vi "HFRR ADV v042.vi"() -> ()   [LabVIEW 2025] (continued)
                  }
                  frame True {
                    n297 = Not(x=w407) -> (.not. x?=w406:bool)
                    n298 = call "ELAPSED TIMER VI - abort test.vi"("TARGET"=60.0, "RESET"=w406, "PAUSE"=FALSE) -> ("ELAPSED INDICATION"=w404:bool)  [unwired: 6 in, 2 out]
                    n299 = case shown="True" w404 {
                      frame False {
                      }
                      frame True {
                        n300 = stacked-sequence {
                          frame #0 {
                            w409 = FALSE
                            n301 = local write "RUN"(w409) -> ()
                            n302 = local write "Auto Start Test"(w409) -> ()
                          }
                          frame #1 {
                            n303 = One Button Dialog(message="Test stopped due to a communication error. Reconnect the C1 and C2 cables.") -> ()  [unwired: 1 in, 1 out]
                          }
                        }
                      }
                    }
                  }
                }
              }
            }
          }
          frame Enabled {
          }
        }
        n304 = Get Date/Time In Seconds() -> (seconds since 1Jan1904=w390:timestamp)
        n305 = Format Into String(format string="%<%I:%M:%S:%p %d:%B:%Y>T", w390) -> (resulting string=→"Time Stamp":string)  [unwired: 2 in, 1 out]
        n306 = local read "Service Password enable"() -> (w382:bool)
        n307 = local read "FILE"() -> (w387:string)
        n308 = call <vilib>:"Trim Whitespace.vi"("string"=w387) -> ("trimmed string"=w386:string)  [unwired: 1 in]
        n309 = String Length(string=w386) -> (length=w385:i32)
        n310 = Greater?(x=w385, y=1) -> (0:w383:bool)
        n311 = case shown="False" w383 {
          tunnel: w382 -> [w411 _]
          frame False {
            n312 = case shown="False" w411 {
              frame True {
                w412 = "Test Start In Service Mode" ("Tip Strip")
                w413 = T19."Enabled" ("Disabled")
                n313 = property on="Auto Start Test" class="Bool (strict)"("DisabledEnum"=w413, "TipStrip"=w412) -> ()  [unwired: 2 in, 2 out]
                n314 = property on="RUN" class="Bool (strict)"("DisabledEnum"=w413, "TipStrip"=w412) -> ()  [unwired: 2 in, 2 out]
              }
              frame False {
                w414 = "Enter File Name to Start Test" ("Tip Strip")
                w415 = T19."Disabled and Grayed Out" ("Disabled")
                n315 = property on="Auto Start Test" class="Bool (strict)"("DisabledEnum"=w415, "TipStrip"=w414) -> ()  [unwired: 2 in, 2 out]
                n316 = property on="RUN" class="Bool (strict)"("DisabledEnum"=w415, "TipStrip"=w414) -> ()  [unwired: 2 in, 2 out]
              }
            }
          }
          frame True {
            w416 = "" ("Tip Strip")
            w417 = T19."Enabled" ("Disabled")
            n317 = property on="Auto Start Test" class="Bool (strict)"("DisabledEnum"=w417, "TipStrip"=w416) -> ()  [unwired: 2 in, 2 out]
            n318 = property on="RUN" class="Bool (strict)"("DisabledEnum"=w417, "TipStrip"=w416) -> ()  [unwired: 2 in, 2 out]
          }
        }
      }
      event "RUN": Value Change {
        n319 = event-data() -> ()  [unwired: 1 in, 6 out]
        n320 = local read "RUN"() -> (w419:bool)
        n321 = case shown="False" w419 {
          frame False {
            n322 = flat-sequence {
              frame #0 {
                n323 = local write "START TEMP"(FALSE ("START TEMP")) -> ()
              }
              frame #1 {
                n324 = Wait (ms)(milliseconds to wait=u32 1500) -> ()  [unwired: 1 out]
              }
              frame #2 {
                n325 = local write "Humidity 2"(TRUE ("Humidity")) -> ()
              }
              frame #3 {
                n326 = local write "Due Write"("VC;0") -> ()
              }
              frame #4 {
                n327 = Wait (ms)(milliseconds to wait=u32 1500) -> ()  [unwired: 1 out]
              }
              frame #5 {
                w429 = T19."Enabled" ("Disabled")
                (unwired) T25."Imaging" ("Main Dashboard Buttons")
                (unwired) T21."Adv Scar" ("Main Tab")
                w431 = "" ("FILE")
                n328 = local write "measured_stroke"(0.0 ("measured_stroke")) -> ()
                n329 = local write "Due Write"("VC;0") -> ()
                n330 = local write "FILE"(w431) -> ()
                n331 = local write "Batch Ref Num :"(w431) -> ()
                n332 = local write "Fuel Discription :"(w431) -> ()
                n333 = local write "Main Tab"(T2."Adv Scar" ("Main Tab")) -> ()
                n334 = local write "Remarks :"(w431) -> ()
                n335 = local write "Main Dashboard Buttons"(T1."Imaging" ("Main Dashboard Buttons")) -> ()
                n336 = local write "TEST FILE NAM,E SAVED"(FALSE ("TEST FILE NAM,E SAVED")) -> ()
                n337 = property on="Stroke ( mm )" class="WFChart (strict)"("History Data"=cluster{"y":dbl, dbl, "y":dbl}[] []) -> ()  [unwired: 2 in, 2 out]
                n338 = property on="Auto Start Test" class="Bool (strict)"("Visible"=TRUE) -> ()  [unwired: 2 in, 2 out]
                n339 = property on="FRICVALZ 2" class="Bool (strict)"("DisabledEnum"=w429) -> ()  [unwired: 2 in, 2 out]
                n340 = property on="FRICVALZ 4" class="Bool (strict)"("DisabledEnum"=w429) -> ()  [unwired: 2 in, 2 out]
                n341 = property on="FRICVALZ 3" class="Bool (strict)"("DisabledEnum"=w429) -> ()  [unwired: 2 in, 2 out]
              }
            }
          }
          frame True {
            n342 = stacked-sequence {
              frame #0 {
                n343 = local write "Due Write"("DAC;200") -> ()
              }
              frame #1 {
                n344 = Wait (ms)(milliseconds to wait=u32 1500) -> ()  [unwired: 1 out]
              }
              frame #2 {
                n345 = local write "Due Write"("DAC;200") -> ()
              }
              frame #3 {
                n346 = Wait (ms)(milliseconds to wait=u32 1500) -> ()  [unwired: 1 out]
              }
              frame #4 {
                n347 = local write "Due Write"("VC;1") -> ()
              }
              frame #5 {
                n348 = Wait (ms)(milliseconds to wait=u32 2000) -> ()  [unwired: 1 out]
              }
              frame #6 {
                n349 = local write "Due Write"("VC;1") -> ()
              }
              frame #7 {
                n350 = Wait (ms)(milliseconds to wait=u32 2000) -> ()  [unwired: 1 out]
              }
              frame #8 {
                w443 = T19."Disabled" ("Disabled")
                n351 = property on="Auto Start Test" class="Bool (strict)"("Visible"=FALSE) -> ()  [unwired: 2 in, 2 out]
                n352 = local write "START TEMP"(TRUE ("START TEMP")) -> ()
                n353 = property on="FRICVALZ 2" class="Bool (strict)"("DisabledEnum"=w443) -> ()  [unwired: 2 in, 2 out]
                n354 = property on="FRICVALZ 4" class="Bool (strict)"("DisabledEnum"=w443) -> ()  [unwired: 2 in, 2 out]
                n355 = property on="FRICVALZ 3" class="Bool (strict)"("DisabledEnum"=w443) -> ()  [unwired: 2 in, 2 out]
              }
            }
          }
        }
      }
      event "run test Calibration": Value Change {
        n356 = event-data() -> ()  [unwired: 1 in, 6 out]
        n357 = local read "run test Calibration"() -> (w445:bool)
        n358 = case shown="True" w445 {
          frame False {
            n359 = flat-sequence {
              frame #0 {
                n360 = local write "START TEMP"(FALSE ("START TEMP")) -> ()
              }
              frame #1 {
                n361 = Wait (ms)(milliseconds to wait=u32 1500) -> ()  [unwired: 1 out]
              }
              frame #2 {
              }
              frame #3 {
                n362 = local write "Due Write"("VC;0") -> ()
              }
              frame #4 {
                n363 = Wait (ms)(milliseconds to wait=u32 1500) -> ()  [unwired: 1 out]
              }
              frame #5 {
                n364 = local write "Due Write"("VC;0") -> ()
                n365 = local write "Friction Force Calibration Result Tab"(enum32{"Calibration Results", "Page 2"}."Calibration Results" ("Friction Force Calibration Result Tab")) -> ()
                n366 = property on="Friction Force Calibration Result Tab" class="TabCtl (strict)"("Visible"=TRUE) -> ()  [unwired: 2 in, 2 out]
              }
            }
          }
          frame True {
            n367 = flat-sequence {
              frame #0 {
                n368 = local write "Due Write"("VC;1") -> ()
              }
              frame #1 {
                n369 = Wait (ms)(milliseconds to wait=u32 2000) -> ()  [unwired: 1 out]
              }
              frame #2 {
                n370 = local write "Due Write"("VC;1") -> ()
              }
              frame #3 {
                n371 = Wait (ms)(milliseconds to wait=u32 2000) -> ()  [unwired: 1 out]
              }
              frame #4 {
                n372 = local write "START TEMP"(TRUE ("START TEMP")) -> ()
                n373 = local write "Friction Force Calibration Result Tab"(enum32{"Calibration Results", "Page 2"}."Calibration Results" ("Friction Force Calibration Result Tab")) -> ()
                n374 = property on="Friction Force Calibration Result Tab" class="TabCtl (strict)"("Visible"=TRUE) -> ()  [unwired: 2 in, 2 out]
              }
            }
          }
        }
      }
      event "Auto": Value Change {
        n375 = event-data() -> ()  [unwired: 1 in, 6 out]
        n376 = stacked-sequence {
          frame #0 {
            n377 = local write "FILE"("") -> ()
          }
          frame #1 {
            n378 = Get Date/Time In Seconds() -> (seconds since 1Jan1904=w465:timestamp)
            n379 = Format Into String(format string="%<%I_%M_%S_%p_%d_%B_%Y>T", w465) -> (resulting string=w464:string)  [unwired: 2 in, 1 out]
            n380 = local write "FILE"(w464) -> ()
          }
        }
        n381 = local read "Auto"() -> (w462:bool)
        n382 = Not(x=w462) -> (.not. x?=w461:bool)
        n383 = local write "Auto"(w461) -> ()
      }
      event "Auto Start Temp": Value Change {
        n384 = event-data() -> ()  [unwired: 1 in, 6 out]
        n385 = local read "Auto Start Test"() -> (w468:bool)
        n386 = case shown="False" w468 {
          frame False {
            n387 = stacked-sequence {
              frame #0 {
                n388 = local write "START TEMP"(FALSE ("START TEMP")) -> ()
              }
              frame #1 {
                n389 = Wait (ms)(milliseconds to wait=u32 2000) -> ()  [unwired: 1 out]
              }
              frame #2 {
                n390 = local write "Due Write"("VC;0") -> ()
              }
              frame #3 {
                n391 = Wait (ms)(milliseconds to wait=u32 2000) -> ()  [unwired: 1 out]
              }
              frame #4 {
                w479 = T19."Enabled" ("Disabled")
                (unwired) T25."Imaging" ("Main Dashboard Buttons")
                w480 = "" ("FILE")
                n392 = local write "Main Tab"(T2."Adv Scar" ("Main Tab")) -> ()
                n393 = local write "measured_stroke"(0.0 ("measured_stroke")) -> ()
                n394 = local write "Main Dashboard Buttons"(T1."Imaging" ("Main Dashboard Buttons")) -> ()
                n395 = property on="RUN" class="Bool (strict)"("Visible"=TRUE) -> ()  [unwired: 2 in, 2 out]
                n396 = local write "Due Write"("VC;0") -> ()
                n397 = local write "Humidity 2"(TRUE ("Humidity")) -> ()
                n398 = local write "TEST FILE NAM,E SAVED"(FALSE ("TEST FILE NAM,E SAVED")) -> ()
                n399 = local write "Fuel Discription :"(w480) -> ()
                n400 = local write "Batch Ref Num :"(w480) -> ()
                n401 = local write "Remarks :"(w480) -> ()
                n402 = local write "FILE"(w480) -> ()
                n403 = property on="FRICVALZ 2" class="Bool (strict)"("DisabledEnum"=w479) -> ()  [unwired: 2 in, 2 out]
                n404 = property on="FRICVALZ 4" class="Bool (strict)"("DisabledEnum"=w479) -> ()  [unwired: 2 in, 2 out]
                n405 = property on="FRICVALZ 3" class="Bool (strict)"("DisabledEnum"=w479) -> ()  [unwired: 2 in, 2 out]
              }
            }
          }
          frame True {
            n406 = stacked-sequence {
              frame #0 {
                n407 = local write "Due Write"("DAC;200") -> ()
              }
              frame #1 {
                n408 = Wait (ms)(milliseconds to wait=u32 1500) -> ()  [unwired: 1 out]
              }
              frame #2 {
                n409 = local write "Due Write"("DAC;200") -> ()
              }
              frame #3 {
                n410 = Wait (ms)(milliseconds to wait=u32 1000) -> ()  [unwired: 1 out]
              }
              frame #4 {
                n411 = local write "Due Write"("VC;1") -> ()
              }
              frame #5 {
                n412 = Wait (ms)(milliseconds to wait=u32 2000) -> ()  [unwired: 1 out]
              }
              frame #6 {
                n413 = local write "Due Write"("VC;1") -> ()
              }
              frame #7 {
                n414 = Wait (ms)(milliseconds to wait=u32 2000) -> ()  [unwired: 1 out]
              }
              frame #8 {
                w491 = T19."Disabled" ("Disabled")
                n415 = property on="RUN" class="Bool (strict)"("Visible"=FALSE) -> ()  [unwired: 2 in, 2 out]
                n416 = property on="FRICVALZ 2" class="Bool (strict)"("DisabledEnum"=w491) -> ()  [unwired: 2 in, 2 out]
                n417 = property on="FRICVALZ 4" class="Bool (strict)"("DisabledEnum"=w491) -> ()  [unwired: 2 in, 2 out]
                n418 = property on="FRICVALZ 3" class="Bool (strict)"("DisabledEnum"=w491) -> ()  [unwired: 2 in, 2 out]
                "START TEMP" <- TRUE
              }
            }
          }
        }
      }
      event "FILE", "USERNAME", "USER ID": Mouse Enter {
        n419 = event-data() -> ()  [unwired: 1 in, 4 out]
        n420 = dll-call lib="kernel32.dll" fn="Wow64DisableWow64FsRedirection"("OldValue"=0) -> (error out=w498:errorcluster, "OldValue"=w496:i32)  [unwired: 4 in, 1 out]
        n421 = call <vilib>:"System Exec.vi"("run minimized? (F)"=TRUE, "error in (no error)"=w498, "command line"="C:\\Program Files\\Common Files\\Microsoft Shared\\Ink\\TabTip.exe") -> ("error out"=w497:errorcluster)  [unwired: 5 in, 3 out]
        n422 = dll-call lib="kernel32.dll" fn="Wow64EnableWow64FsRedirection"(error in=w497, "OldValue"=w496) -> ()  [unwired: 4 in, 2 out]
      }
      event "EDIT": Value Change {
        n423 = event-data() -> ()  [unwired: 1 in, 6 out]
        n424 = local read "EDIT"() -> (w499:bool)
        n425 = case shown="False" w499 {
          frame False {
            n426 = control-ref of="This VI"() -> (w516:refnum<vi>)
            n427 = property class="VI"(reference=w516) -> (reference out=w507:refnum<vi>, error out=w511:errorcluster, "Panel"=w515:refnum<vi>)  [unwired: 1 in]
            n428 = property class="Pnl"(reference=w515, error in=w511) -> (reference out=w509:refnum<vi>, error out=w512:errorcluster, "Panes[]"=w514:refnum<vi>[])
            n429 = for {
              tunnel: w514 -> [w522] mode=indexing
              tunnel: T24."Always Off" ("Horizontal Scrollbar Visibility") -> [w521]
              tunnel: w512 -> [w518]
              tunnel: [w517] -> w510
              n430 = property class="Pane"(reference=w522, error in=w518, "HorizScrollbarVisibility"=w521) -> (reference out=w519:refnum<vi>, error out=w520:errorcluster)
              n431 = Close Reference(reference=w519, error in (no error)=w520) -> (error out=w517:errorcluster)
            }
            n432 = Close Reference(reference=w509, error in (no error)=w510) -> (error out=w508:errorcluster)
            n433 = Close Reference(reference=w507, error in (no error)=w508) -> (error out=w502:errorcluster)
            "error out 7" <- w502
            n434 = call <vilib>:"Clear Errors.vi"("error in (no error)"=w502) -> ("error out"=w501:errorcluster)  [unwired: 5 in, 1 out]
            n435 = local write "Service Password enable"(FALSE ("Service Password enable")) -> ()
            n436 = call <userlib>:"Fit VI window to Largest Dec.vi"("error in (no error)"=w501, "border spacing (2 px)"=1) -> ("error out"=w506:errorcluster, "dup VI Ref"=w504:refnum<vi>)  [unwired: 4 in]
            n437 = invoke on="Invoke Node" class="VI" method="FP.Run-Time Position.Maximized"(reference=w504, error in=w506) -> (error out=w505:errorcluster)  [unwired: 2 in, 3 out]
            n438 = call <vilib>:"Clear Errors.vi"("error in (no error)"=w505) -> ()  [unwired: 5 in, 2 out]
          }
          frame True {
          }
        }
      }
      event "Heater Button": Value Change {
        n439 = event-data() -> ()  [unwired: 1 in, 6 out]
        n440 = local read "Heater Button"() -> (w523:bool)
        n441 = case shown="True" w523 {
          frame True {
            n442 = stacked-sequence {
              frame #0 {
                n443 = Wait (ms)(milliseconds to wait=u32 1500) -> ()  [unwired: 1 out]
              }
              frame #1 {
                n444 = local read "Set Temp"() -> (w525:dbl)
                n445 = Number To Fractional String(number=w525, precision (6)=i16 2) -> (F-format string=w528:string)  [unwired: 2 in]
                n446 = Concatenate Strings("ST;" ("Command"), w528) -> (w527:string)
                n447 = local write "Due Write"(w527) -> ()
              }
              frame #2 {
                n448 = Wait (ms)(milliseconds to wait=u32 1500) -> ()  [unwired: 1 out]
              }
              frame #3 {
                n449 = local write "Due Write"("HE;1" ("Command")) -> ()
              }
              frame #4 {
                n450 = Wait (ms)(milliseconds to wait=u32 1500) -> ()  [unwired: 1 out]
              }
              frame #5 {
                n451 = stacked-sequence {
                  frame #0 {
                    n452 = Wait (ms)(milliseconds to wait=u32 1500) -> ()  [unwired: 1 out]
                  }
                  frame #1 {
                    n453 = local read "Set Temp"() -> (w534:dbl)
                    n454 = Number To Fractional String(number=w534, precision (6)=i16 2) -> (F-format string=w537:string)  [unwired: 2 in]
                    n455 = Concatenate Strings("ST;" ("Command"), w537) -> (w536:string)
                    n456 = local write "Due Write"(w536) -> ()
                  }
                  frame #2 {
                    n457 = Wait (ms)(milliseconds to wait=u32 1500) -> ()  [unwired: 1 out]
                  }
                  frame #3 {
                    n458 = local write "Due Write"("HE;1" ("Command")) -> ()
                  }
                  frame #4 {
                    n459 = Wait (ms)(milliseconds to wait=u32 1500) -> ()  [unwired: 1 out]
                  }
                }
              }
            }
          }
          frame False {
            n460 = stacked-sequence {
              frame #0 {
                n461 = Wait (ms)(milliseconds to wait=u32 1500) -> ()  [unwired: 1 out]
              }
              frame #1 {
                n462 = Concatenate Strings("ST;" ("Command"), "0" ("string")) -> (w544:string)
                n463 = local write "Due Write"(w544) -> ()
              }
              frame #2 {
                n464 = Wait (ms)(milliseconds to wait=u32 1500) -> ()  [unwired: 1 out]
              }
              frame #3 {
                n465 = local write "Due Write"("HE;0" ("Command")) -> ()
              }
              frame #4 {
                n466 = Wait (ms)(milliseconds to wait=u32 1500) -> ()  [unwired: 1 out]
              }
            }
          }
        }
      }
      event "Headen Service Button": Value Change {
        n467 = event-data() -> ()  [unwired: 1 in, 6 out]
        n468 = local read "Headen Service Button"() -> (w549:bool)
        n469 = case shown="True" w549 {
          frame False {
            n470 = property on="Password 3" class="Clust (strict)"("Visible"=FALSE) -> ()  [unwired: 2 in, 2 out]
            n471 = property on="Service Password Log" class="Str"("Visible"=FALSE) -> ()  [unwired: 2 in, 2 out]
          }
          frame True {
            n472 = property on="Password 3" class="Clust (strict)"("Visible"=TRUE) -> ()  [unwired: 2 in, 2 out]
            n473 = property on="Service Password Log" class="Str"("Visible"=TRUE) -> ()  [unwired: 2 in, 2 out]
          }
        }
      }
      event "Password 3.Service Password": Value Change {
        n474 = event-data() -> ()  [unwired: 1 in, 6 out]
        n475 = Unbundle By Name("Password 3") -> ("Service Password"=w556:string)
        n476 = call <vilib>:"Trim Whitespace.vi"("string"=w556) -> ("trimmed string"=w554:string)  [unwired: 1 in]
        n477 = Equal?(x=w554, y="Service@123") -> (x = y?=w555:bool)
        n478 = case shown="False" w555 {
          selector: w555 -> [w559 w561]
          frame False {
            n479 = local write "Service Password enable"(w559) -> ()
            n480 = property on="Service Password Log" class="Str"("Visible"=TRUE) -> ()  [unwired: 2 in, 2 out]
          }
          frame True {
            n481 = property on="Service Password Log" class="Str"("Visible"=FALSE) -> ()  [unwired: 2 in, 2 out]
            "Service Password enable" <- w561
          }
        }
      }
      event "Sign In": Value Change {
        w563 = FALSE ("Visible")
        n482 = event-data() -> ()  [unwired: 1 in, 6 out]
        n483 = property on="About" class="Clust (strict)"("Visible"=w563) -> ()  [unwired: 2 in, 2 out]
        n484 = property on="Password 3" class="Clust (strict)"("Visible"=w563) -> ()  [unwired: 2 in, 2 out]
        n485 = property on="Service Password Log" class="Str"("Visible"=FALSE) -> ()  [unwired: 2 in, 2 out]
      }
      event "Info": Value Change {
        n486 = event-data() -> ()  [unwired: 1 in, 6 out]
        n487 = local read "Info"() -> (w565:bool)
        n488 = case shown="False" w565 {
          frame False {
            n489 = property on="About" class="Clust (strict)"("Visible"=FALSE) -> ()  [unwired: 2 in, 2 out]
          }
          frame True {
            n490 = property on="About" class="Clust (strict)"("Visible"=TRUE) -> ()  [unwired: 2 in, 2 out]
          }
        }
      }
      event "Calibration": Value Change {
        n491 = event-data() -> ()  [unwired: 1 in, 6 out]
        n492 = local read "Calibration"() -> (w569:bool)
        n493 = case shown="False" w569 {
          frame False {
            n494 = property on="Calibration 2" class="TabCtl (strict)"("Visible"=FALSE) -> ()  [unwired: 2 in, 2 out]
            n495 = local write "Cal Password"("" ("Cal Password")) -> ()
          }
          frame True {
            n496 = property on="Calibration 2" class="TabCtl (strict)"("Visible"=TRUE) -> ()  [unwired: 2 in, 2 out]
            n497 = local write "Cal Password"("" ("Cal Password")) -> ()
          }
        }
        n498 = property on="Wrong Password" class="Str"("Visible"=FALSE) -> ()  [unwired: 2 in, 2 out]
      }
      event "Cal Password": Value Change {
        n499 = event-data() -> ()  [unwired: 1 in, 6 out]
        n500 = local read "Cal Password"() -> (w577:string)
        n501 = call <vilib>:"Trim Whitespace.vi"("string"=w577) -> ("trimmed string"=w576:string)  [unwired: 1 in]
        n502 = Equal?(x=w576, y="Cal@321") -> (x = y?=w574:bool)
        n503 = case shown="True" w574 {
          frame False {
            n504 = property on="Wrong Password" class="Str"("Visible"=TRUE) -> ()  [unwired: 2 in, 2 out]
          }
          frame True {
            n505 = property on="Wrong Password" class="Str"("Visible"=FALSE) -> ()  [unwired: 2 in, 2 out]
            n506 = local write "Main Tab"(T2."About" ("Main Tab")) -> ()
            n507 = local write "Cal Password"("" ("Cal Password")) -> ()
            n508 = local write "Main Dashboard Buttons"(T1."About" ("Main Dashboard Buttons")) -> ()
            n509 = property on="Calibration 2" class="TabCtl (strict)"("Visible"=FALSE) -> ()  [unwired: 2 in, 2 out]
            n510 = local write "Calibration"(FALSE ("Calibration")) -> ()
          }
        }
      }
      event "Calibration Selection": Value Change {
        n511 = event-data() -> ()  [unwired: 1 in, 6 out]
        n512 = local read "Calibration Selection"() -> (w586:T8)
        n513 = case shown="\"Stroke Calibration\"" w586 {
          tunnel: [T7."Stroke" ("Main Calibration Tab") T7."Friction" ("Main Calibration Tab") T7."Main" ("Main Calibration Tab") T7."Temperature" ("Main Calibration Tab")] -> w585
          frame "Stroke Calibration" {
          }
          frame "Friction Force Calibration" {
          }
          frame Default {
          }
          frame "Temperature Calibration" {
          }
        }
        n514 = local write "Main Calibration Tab"(w585) -> ()
      }
      event "Back Stroke": Value Change {
        n515 = event-data() -> ()  [unwired: 1 in, 6 out]
        n516 = local write "Main Stroke Tab"(T9."Step 1" ("Main Stroke Tab")) -> ()
        n517 = local write "Main Calibration Tab"(T7."Main" ("Main Calibration Tab")) -> ()
        n518 = local write "Back Stroke"(FALSE ("Back Stroke")) -> ()
        n519 = local write "Calibration Selection"(T8."Default" ("Calibration Selection")) -> ()
      }
      event "Step 2 Back": Value Change {
        n520 = event-data() -> ()  [unwired: 1 in, 6 out]
        n521 = local write "Main Stroke Tab"(T9."Step 1" ("Main Stroke Tab")) -> ()
        n522 = local write "Step 2 Back"(FALSE ("Back Stroke")) -> ()
        n523 = local write "Calibration Selection"(T8."Default" ("Calibration Selection")) -> ()
      }
      event "Step 3 Back": Value Change {
        n524 = event-data() -> ()  [unwired: 1 in, 6 out]
        n525 = local write "Main Stroke Tab"(T9."Step 2" ("Main Stroke Tab")) -> ()
        n526 = local write "Step 3 Back"(FALSE ("Back Stroke")) -> ()
        n527 = local write "Calibration Selection"(T8."Default" ("Calibration Selection")) -> ()
      }
      event "Step 4 Back": Value Change {
        n528 = event-data() -> ()  [unwired: 1 in, 6 out]
        n529 = local write "Main Stroke Tab"(T9."Step 3" ("Main Stroke Tab")) -> ()
        n530 = local write "Step 4 Back"(FALSE ("Back Stroke")) -> ()
        n531 = local write "Calibration Selection"(T8."Default" ("Calibration Selection")) -> ()
      }
      event "Step 5 Back": Value Change {
        n532 = event-data() -> ()  [unwired: 1 in, 6 out]
        n533 = local write "Main Stroke Tab"(T9."Step 4" ("Main Stroke Tab")) -> ()
        n534 = local write "Step 5 Back"(FALSE ("Back Stroke")) -> ()
        n535 = local write "Calibration Selection"(T8."Default" ("Calibration Selection")) -> ()
      }
      event "Step 6 Back": Value Change {
        n536 = event-data() -> ()  [unwired: 1 in, 6 out]
        n537 = local write "Main Stroke Tab"(T9."Step 5" ("Main Stroke Tab")) -> ()
        n538 = local write "Step 6 Back"(FALSE ("Back Stroke")) -> ()
        n539 = local write "Calibration Selection"(T8."Default" ("Calibration Selection")) -> ()
      }
      event "Back Stroke step 7": Value Change {
        n540 = event-data() -> ()  [unwired: 1 in, 6 out]
        n541 = local write "Main Stroke Tab"(T9."Step 5" ("Main Stroke Tab")) -> ()
        n542 = local write "Back Stroke step 7"(FALSE ("Back Stroke")) -> ()
        n543 = local write "Calibration Selection"(T8."Default" ("Calibration Selection")) -> ()
      }
      event "Back Stroke step 8": Value Change {
        n544 = event-data() -> ()  [unwired: 1 in, 6 out]
        n545 = local write "Main Stroke Tab"(T9."Step 7" ("Main Stroke Tab")) -> ()
        n546 = local write "Back Stroke step 8"(FALSE ("Back Stroke")) -> ()
        n547 = local write "Calibration Selection"(T8."Default" ("Calibration Selection")) -> ()
      }
      event "Back Stroke 8": Value Change {
        n548 = event-data() -> ()  [unwired: 1 in, 6 out]
        n549 = local write "MOVE CARRIAGE TO"(1.0 ("MOVE CARRIAGE TO")) -> ()
        n550 = local write "Main Stroke Tab"(T9."Step 1" ("Main Stroke Tab")) -> ()
        n551 = local write "Calibration Selection"(T8."Default" ("Calibration Selection")) -> ()
        n552 = local write "Back Stroke 8"(FALSE ("Back Stroke 8")) -> ()
      }
      event "Continue Stroke": Value Change {
        n553 = event-data() -> ()  [unwired: 1 in, 6 out]
        n554 = local write "Main Stroke Tab"(T9."Step 2" ("Main Stroke Tab")) -> ()
        n555 = local write "Continue Stroke"(FALSE ("Continue Stroke")) -> ()
      }
      event "Continue Stroke step 2": Value Change {
        n556 = event-data() -> ()  [unwired: 1 in, 6 out]
        n557 = local write "Main Stroke Tab"(T9."Step 3" ("Main Stroke Tab")) -> ()
        n558 = local write "Continue Stroke step 2"(FALSE ("Continue Stroke")) -> ()
      }
      event "Continue Stroke step 3": Value Change {
        n559 = event-data() -> ()  [unwired: 1 in, 6 out]
        n560 = local write "Main Stroke Tab"(T9."Step 4" ("Main Stroke Tab")) -> ()
        n561 = local write "Continue Stroke step 3"(FALSE ("Continue Stroke")) -> ()
      }
      event "Continue Stroke step 4": Value Change {
        n562 = event-data() -> ()  [unwired: 1 in, 6 out]
        n563 = local write "Main Stroke Tab"(T9."Step 5" ("Main Stroke Tab")) -> ()
        n564 = local write "Continue Stroke step 4"(FALSE ("Continue Stroke")) -> ()
      }
      event "Continue Stroke step 5": Value Change {
        n565 = event-data() -> ()  [unwired: 1 in, 6 out]
        n566 = local write "Main Stroke Tab"(T9."Step 7" ("Main Stroke Tab")) -> ()
        n567 = local write "Continue Stroke step 5"(FALSE ("Continue Stroke")) -> ()
      }
      event "Continue Stroke step 6": Value Change {
        n568 = event-data() -> ()  [unwired: 1 in, 6 out]
        n569 = local write "Main Stroke Tab"(T9."Step 7" ("Main Stroke Tab")) -> ()
        n570 = local write "Continue Stroke step 6"(FALSE ("Continue Stroke")) -> ()
      }
      event "Continue Stroke step 7": Value Change {
        w634 = FALSE ("0.2mm")
        n571 = event-data() -> ()  [unwired: 1 in, 6 out]
        n572 = local write "0.4 mm"(w634) -> ()
        n573 = local write "0.6 mm"(w634) -> ()
        n574 = local write "1.0 mm"(w634) -> ()
        n575 = local write "1.2 mm"(w634) -> ()
        n576 = local write "0.2 2"(w634) -> ()
        n577 = local write "0.4 2"(w634) -> ()
        n578 = local write "0.6 2"(w634) -> ()
        n579 = local write "0.8 2"(w634) -> ()
        n580 = local write "1.0 2"(w634) -> ()
        n581 = local write "1.2"(w634) -> ()
        n582 = local write "0.2mm"(w634) -> ()
        n583 = local write "0.8mm"(w634) -> ()
        n584 = local write "Main Stroke Tab"(T9."Step 8" ("Main Stroke Tab")) -> ()
        n585 = local write "Continue Stroke step 7"(FALSE ("Continue Stroke")) -> ()
        n586 = local write "Stroke Test Complete"(T10."Test Progress" ("Stroke Test Complete")) -> ()
        "Position Measurment Temp" <- 4.0 ("Position Measurment Temp")
        "Calibration Tare" <- TRUE ("Calibration Tare")
        "MOVE CARRIAGE TO" <- 1.0 ("MOVE CARRIAGE TO")
      }
      event "Continue Stroke step 8": Value Change {
        n587 = event-data() -> ()  [unwired: 1 in, 6 out]
        n588 = local read "LVDT STROKE  Calibration"() -> (w639:dbl)
        n589 = local read "Position Measurment Temp"() -> (w640:dbl)
        n590 = case shown="7" w640 {
          selector: w640 -> [w645 w650 w655 w660 _ w668 w671 w672]
          tunnel: w639 -> [w641 w646 w651 w656 w662 w665 _ _]
          frame 0, Default {
            w643 = TRUE ("0.2mm")
            n591 = Increment(x=w645) -> (x+1=w644:i32)
            n592 = local write "Position Measurment Temp"(w644) -> ()
            n593 = local write "0.2mm"(w643) -> ()
            n594 = local write "0.2 2"(w643) -> ()
            n595 = local write "MOVE CARRIAGE TO"(1.0 ("MOVE CARRIAGE TO")) -> ()
            "Calibration 0.2" <- w641
          }
          frame 1 {
            w648 = TRUE ("0.4 mm")
            n596 = Increment(x=w650) -> (x+1=w649:i32)
            n597 = local write "Calibration 0.4"(w646) -> ()
            n598 = local write "Position Measurment Temp"(w649) -> ()
            n599 = local write "0.4 mm"(w648) -> ()
            n600 = local write "MOVE CARRIAGE TO"(0.6 ("MOVE CARRIAGE TO")) -> ()
            n601 = local write "0.4 2"(w648) -> ()
          }
          frame 2 {
            w653 = TRUE ("0.6 mm")
            n602 = Increment(x=w655) -> (x+1=w654:i32)
            n603 = local write "Calibration 0.6"(w651) -> ()
            n604 = local write "Position Measurment Temp"(w654) -> ()
            n605 = local write "0.6 2"(w653) -> ()
            n606 = local write "0.6 mm"(w653) -> ()
            n607 = local write "MOVE CARRIAGE TO"(0.8 ("MOVE CARRIAGE TO")) -> ()
          }
          frame 3 {
            w657 = TRUE ("0.6 mm")
            n608 = Increment(x=w660) -> (x+1=w659:i32)
            n609 = local write "Position Measurment Temp"(w659) -> ()
            n610 = local write "MOVE CARRIAGE TO"(1.0 ("MOVE CARRIAGE TO")) -> ()
            n611 = local write "0.8mm"(w657) -> ()
            n612 = local write "0.8 2"(w657) -> ()
            "Calibration 0.8" <- w656
          }
          frame 4 {
            w663 = TRUE ("0.6 mm")
            n613 = local write "Position Measurment Temp"(6.0 ("Position Measurment Temp")) -> ()
            n614 = local write "MOVE CARRIAGE TO"(1.0 ("MOVE CARRIAGE TO")) -> ()
            n615 = local write "1.0 mm"(w663) -> ()
            n616 = local write "1.0 2"(w663) -> ()
            "Calibration 1.0" <- w662
          }
          frame 5 {
            w666 = TRUE ("0.6 mm")
            n617 = Increment(x=w668) -> (x+1=w667:i32)
            n618 = local write "Position Measurment Temp"(w667) -> ()
            n619 = local write "1.2 mm"(w666) -> ()
            n620 = local write "1.2"(w666) -> ()
            "Calibration 1.2" <- w665
          }
          frame 6 {
            n621 = Increment(x=w671) -> (x+1=w670:i32)
            n622 = local write "Position Measurment Temp"(w670) -> ()
            n623 = local write "Stroke Test Complete"(T10."Stroke Points Completed" ("Stroke Test Complete")) -> ()
          }
          frame 7 {
            n624 = stacked-sequence {
              tunnel: w672 -> [w673 _ _]
              frame #0 {
                n625 = Increment(x=w673) -> (x+1=w674:i32)
                n626 = local write "Main Stroke Tab"(T9."Step 9" ("Main Stroke Tab")) -> ()
                n627 = local write "Position Measurment Temp"(w674) -> ()
                n628 = Insert Into Array(array=dbl[] [], new element #1=0.2 ("new element/subarray"), new element #2=0.4 ("new element/subarray"), new element #3=0.6 ("new element/subarray"), new element #4=0.8 ("new element/subarray"), new element #5=1.0 ("new element/subarray"), new element #6=1.2 ("new element/subarray")) -> (→"1D stroke":dbl[])  [unwired: 1 in]
                n629 = local read "Calibration 0.2"() -> (w681:dbl)
                n630 = local read "Calibration 0.4"() -> (w680:dbl)
                n631 = local read "Calibration 0.6"() -> (w679:dbl)
                n632 = local read "Calibration 0.8"() -> (w678:dbl)
                n633 = local read "Calibration 1.0"() -> (w677:dbl)
                n634 = local read "Calibration 1.2"() -> (w676:dbl)
                n635 = Insert Into Array(array=dbl[] [], new element #1=w681, new element #2=w680, new element #3=w679, new element #4=w678, new element #5=w677, new element #6=w676) -> (→"Calibrated Voltage Value":dbl[])  [unwired: 1 in]
              }
              frame #1 {
                n636 = local read "calibration values"() -> (w704:dbl[])
                n637 = local read "Calibrated Voltage Value"() -> (w706:dbl[])
                n638 = Index Array(array=w704, index #1=1 ("index"), index #2=3 ("index"), index #3=5 ("index"), index #4=7 ("index"), index #5=9 ("index"), index #6=11 ("index")) -> (element #1=w697:dbl, element #2=w696:dbl, element #3=w695:dbl, element #4=w694:dbl, element #5=w693:dbl, element #6=w692:dbl)
                n639 = local read "1D stroke"() -> (w707:dbl[])
                n640 = for {
                  tunnel: [w716] -> w705 mode=indexing
                  tunnel: w707 -> [w715] mode=indexing
                  tunnel: w706 -> [w714] mode=indexing
                  tunnel: w697 -> [w713]
                  tunnel: w696 -> [w712]
                  tunnel: w695 -> [w711]
                  tunnel: w694 -> [w710]
                  tunnel: w693 -> [w709]
                  tunnel: w692 -> [w708]
                  n641 = formula code="if (stroke == 0.2)\n{\n    if ((voltage >= REF_02 - 0.2) && (voltage <= REF_02 + 0.2))\n        status = 1;\n    else\n        status = 0;\n}\nelse if (stroke == 0.4)\n{\n    if ((voltage >= REF_04 - 0.2) && (voltage <= REF_04 + 0.2))\n        status = 1;\n    else\n        status = 0;\n}\nelse if (stroke == 0.6)\n{\n    if ((voltage >= REF_06 - 0.2) && (voltage <= REF_06 + 0.2))\n        status = 1;\n    else\n        status = 0;\n}\nelse if (stroke == 0.8)\n{\n    if ((voltage >= REF_08 - 0.2) && (voltage <= REF_08 + 0.2))\n        status = 1;\n    else\n        status = 0;\n}\nelse if (stroke == 1.0)\n{\n    if ((voltage >= REF_10 - 0.4) && (voltage <= REF_10 + 0.4))\n        status = 1;\n    else\n        status = 0;\n}\nelse if (stroke == 1.2)\n{\n    if ((voltage >= REF_12 - 0.2) && (voltage <= REF_12 + 0.2))\n        status = 1;\n    else\n        status = 0;\n}\nelse\n{\n    status = 0;\n}"("stroke"=w715, "voltage"=w714, "REF_02"=w713, "REF_04"=w712, "REF_06"=w711, "REF_08"=w710, "REF_10"=w709, "REF_12"=w708) -> ("status"=w716:dbl)
                }
                "Status" <- w705
              }
              frame #2 {
                w723 = 1.0
                n642 = local read "Status"() -> (w730:dbl[])
                n643 = Index Array(array=w730) -> (element #1=w729:dbl, element #2=w728:dbl, element #3=w727:dbl, element #4=w726:dbl, element #5=w725:dbl, element #6=w724:dbl)  [unwired: 6 in]
                n644 = Equal?(x=w728, y=w723) -> (x = y?=w721:bool)
                n645 = Equal?(x=w727, y=w723) -> (x = y?=w720:bool)
                n646 = Equal?(x=w726, y=w723) -> (x = y?=w719:bool)
                n647 = Equal?(x=w725, y=w723) -> (x = y?=w718:bool)
                n648 = Equal?(x=w724, y=w723) -> (x = y?=w717:bool)
                n649 = Equal?(x=w729, y=w723) -> (x = y?=w722:bool)
                n650 = case shown="True" w722 {
                  selector: w722 -> [w741 w742]
                  frame True {
                    n651 = local write "Point 1 - 0.2 mm"(w741) -> ()
                    n652 = property on="Point 1 - 0.2 mm" class="Bool"("Caption.Visible"=w741) -> ()  [unwired: 2 in, 2 out]
                  }
                  frame False {
                    n653 = local write "Point 1 - 0.2 mm"(w742) -> ()
                    n654 = property on="Point 1 - 0.2 mm" class="Bool"("Caption.Visible"=w742) -> ()  [unwired: 2 in, 2 out]
                  }
                }
                n655 = case shown="True" w721 {
                  selector: w721 -> [w739 w740]
                  frame True {
                    n656 = local write "Point 2 - 0.4 mm"(w739) -> ()
                    n657 = property on="Point 2 - 0.4 mm" class="Bool"("Caption.Visible"=w739) -> ()  [unwired: 2 in, 2 out]
                  }
                  frame False {
                    n658 = local write "Point 2 - 0.4 mm"(w740) -> ()
                    n659 = property on="Point 2 - 0.4 mm" class="Bool"("Caption.Visible"=w740) -> ()  [unwired: 2 in, 2 out]
                  }
                }
                n660 = case shown="True" w718 {
                  selector: w718 -> [w733 w734]
                  frame True {
                    n661 = local write "Point 5 - 1.0 mm"(w733) -> ()
                    n662 = property on="Point 5 - 1.0 mm" class="Bool"("Caption.Visible"=w733) -> ()  [unwired: 2 in, 2 out]
                  }
                  frame False {
                    n663 = local write "Point 5 - 1.0 mm"(w734) -> ()
                    n664 = property on="Point 5 - 1.0 mm" class="Bool"("Caption.Visible"=w734) -> ()  [unwired: 2 in, 2 out]
                  }
                }
                n665 = case shown="True" w720 {
                  selector: w720 -> [w737 w738]
                  frame True {
                    n666 = local write "Point 3 - 0.6 mm"(w737) -> ()
                    n667 = property on="Point 3 - 0.6 mm" class="Bool"("Caption.Visible"=w737) -> ()  [unwired: 2 in, 2 out]
                  }
                  frame False {
                    n668 = local write "Point 3 - 0.6 mm"(w738) -> ()
                    n669 = property on="Point 3 - 0.6 mm" class="Bool"("Caption.Visible"=w738) -> ()  [unwired: 2 in, 2 out]
                  }
                }
                n670 = case shown="True" w719 {
                  selector: w719 -> [w735 w736]
                  frame True {
                    n671 = local write "Point 4 - 0.8 mm"(w735) -> ()
                    n672 = property on="Point 4 - 0.8 mm" class="Bool"("Caption.Visible"=w735) -> ()  [unwired: 2 in, 2 out]
                  }
                  frame False {
                    n673 = local write "Point 4 - 0.8 mm"(w736) -> ()
                    n674 = property on="Point 4 - 0.8 mm" class="Bool"("Caption.Visible"=w736) -> ()  [unwired: 2 in, 2 out]
                  }
                }
                n675 = case shown="True" w717 {
                  selector: w717 -> [w731 w732]
                  frame True {
                    n676 = local write "Point 6 - 1.2 mm"(w731) -> ()
                    n677 = property on="Point 6 - 1.2 mm" class="Bool"("Caption.Visible"=w731) -> ()  [unwired: 2 in, 2 out]
                  }
                  frame False {
                    n678 = local write "Point 6 - 1.2 mm"(w732) -> ()
                    n679 = property on="Point 6 - 1.2 mm" class="Bool"("Caption.Visible"=w732) -> ()  [unwired: 2 in, 2 out]
                  }
                }
              }
            }
          }
        }
      }
      event "Accept & Save": Value Change {
        n680 = event-data() -> ()  [unwired: 1 in, 6 out]
        n681 = flat-sequence {
          frame #0 {
            n682 = Get Date/Time In Seconds() -> (seconds since 1Jan1904=w745:timestamp)
            n683 = Format Into String(format string="%<%I:%M:%S:%p %d:%B:%Y>T", w745) -> (resulting string=w743:string)  [unwired: 2 in, 1 out]
            n684 = local write "STROKE CALIBRATION"(w743) -> ()
          }
          frame #1 {
            n685 = local write "Save Button"(TRUE ("Save Button")) -> ()
          }
          frame #2 {
            n686 = local write "MOVE CARRIAGE TO"(1.0 ("MOVE CARRIAGE TO")) -> ()
            n687 = local write "Main Calibration Tab"(T7."Main" ("Main Calibration Tab")) -> ()
            n688 = local write "Main Stroke Tab"(T9."Step 1" ("Main Stroke Tab")) -> ()
            n689 = local write "Calibration Selection"(T8."Default" ("Calibration Selection")) -> ()
            n690 = local write "Back Stroke 8"(FALSE ("Back Stroke 8")) -> ()
          }
        }
      }
      event "TEMPERATURE STEP Back 1", "TEMPERATURE STEP Back air Temp": Value Change {
        n691 = event-data() -> ()  [unwired: 1 in, 6 out]
        n692 = stacked-sequence {
          frame #0 {
            n693 = local write "Main Calibration Tab"(T7."Main" ("Main Calibration Tab")) -> ()
            n694 = local write "Temperature Selection"(T13."Default" ("Temperature Selection")) -> ()
          }
          frame #1 {
            n695 = Wait (ms)(milliseconds to wait=u32 1000) -> ()  [unwired: 1 out]
            n696 = local write "Calibration Selection"(T8."Default" ("Calibration Selection")) -> ()
          }
          frame #2 {
            n697 = local write "Due Write"("CAL;END" ("Command")) -> ()
          }
          frame #3 {
            n698 = Wait (ms)(milliseconds to wait=u32 2000) -> ()  [unwired: 1 out]
          }
          frame #4 {
            n699 = local write "Due Write"("CAL;END" ("Command")) -> ()
          }
        }
      }
      event "Temperature Continue Step 1": Value Change {
        n700 = event-data() -> ()  [unwired: 1 in, 6 out]
        n701 = stacked-sequence {
          frame #0 {
            n702 = Wait (ms)(milliseconds to wait=u32 1500) -> ()  [unwired: 1 out]
          }
          frame #1 {
            n703 = local write "Due Write"("CAL;START" ("Command")) -> ()
          }
          frame #2 {
            n704 = Wait (ms)(milliseconds to wait=u32 1500) -> ()  [unwired: 1 out]
          }
          frame #3 {
            n705 = local write "Due Write"("CAL;START" ("Command")) -> ()
          }
          frame #4 {
            n706 = Wait (ms)(milliseconds to wait=u32 2000) -> ()  [unwired: 1 out]
          }
          frame #5 {
          }
          frame #6 {
            n707 = Wait (ms)(milliseconds to wait=u32 2000) -> ()  [unwired: 1 out]
          }
          frame #7 {
            # "CAL;A1;<true_T>"
            n708 = local write "Due Write"("CAL;A1;0" ("Command")) -> ()
          }
          frame #8 {
            n709 = local write "Tab Control 4"(T12."Step 2" ("Tab Control 4")) -> ()
          }
        }
      }
      event "Temperature Continue Step air Step 1": Value Change {
        n710 = event-data() -> ()  [unwired: 1 in, 6 out]
        n711 = stacked-sequence {
          frame #0 {
            n712 = Wait (ms)(milliseconds to wait=u32 1500) -> ()  [unwired: 1 out]
          }
          frame #1 {
            n713 = local write "Due Write"("CAL;START" ("Command")) -> ()
          }
          frame #2 {
            n714 = Wait (ms)(milliseconds to wait=u32 1500) -> ()  [unwired: 1 out]
          }
          frame #3 {
            n715 = local write "Due Write"("CAL;START" ("Command")) -> ()
          }
          frame #4 {
            n716 = Wait (ms)(milliseconds to wait=u32 2000) -> ()  [unwired: 1 out]
          }
          frame #5 {
          }
          frame #6 {
            n717 = Wait (ms)(milliseconds to wait=u32 2000) -> ()  [unwired: 1 out]
          }
          frame #7 {
            # "CAL;A1;<true_T>"
            n718 = local write "Due Write"("CAL;A1;0" ("Command")) -> ()
          }
          frame #8 {
            n719 = local write "Tab Control 4"(T12."Air Step 2" ("Tab Control 4")) -> ()
          }
        }
      }
      event "Temperature Selection": Value Change {
        n720 = event-data() -> ()  [unwired: 1 in, 6 out]
        n721 = local read "Temperature Selection"() -> (w775:T13)
        n722 = case shown="\"Sample Temperature\"" w775 {
          frame "Air Temperature" {
            n723 = local write "Tab Control 4"(T12."Air Step 1" ("Tab Control 4")) -> ()
          }
          frame "Sample Temperature" {
            n724 = local write "Tab Control 4"(T12."Step 1" ("Tab Control 4")) -> ()
          }
          frame "Default", Default {
          }
        }
      }
      event "Temperature Continue Step 2": Value Change {
        n725 = event-data() -> ()  [unwired: 1 in, 6 out]
        n726 = stacked-sequence {
          frame #0 {
            n727 = stacked-sequence {
              frame #0 {
                n728 = Wait (ms)(milliseconds to wait=u32 1500) -> ()  [unwired: 1 out]
              }
              frame #1 {
                # "CAL;A1;<true_T>"
                n729 = local read "Sensor value"() -> (→"Sample 0deg temp":dbl)
                n730 = local write "Due Write"("CAL;A1;0" ("Command")) -> ()
              }
              frame #2 {
                n731 = Wait (ms)(milliseconds to wait=u32 1500) -> ()  [unwired: 1 out]
              }
              frame #3 {
                # "CAL;A1;<true_T>"
                n732 = local write "Due Write"("CAL;A1;0" ("Command")) -> ()
              }
              frame #4 {
              }
            }
          }
          frame #1 {
            n733 = local write "Tab Control 4"(T12."Step 3" ("Tab Control 4")) -> ()
          }
        }
      }
      event "Temperature Continue Air Step 2": Value Change {
        n734 = event-data() -> ()  [unwired: 1 in, 6 out]
        n735 = stacked-sequence {
          frame #0 {
            n736 = stacked-sequence {
              frame #0 {
                n737 = Wait (ms)(milliseconds to wait=u32 1000) -> ()  [unwired: 1 out]
              }
              frame #1 {
                # "CAL;A1;<true_T>"
                n738 = local write "Due Write"("CAL;A1;0" ("Command")) -> ()
              }
              frame #2 {
                n739 = Wait (ms)(milliseconds to wait=u32 1000) -> ()  [unwired: 1 out]
              }
              frame #3 {
                # "CAL;A1;<true_T>"
                n740 = local write "Due Write"("CAL;A1;0" ("Command")) -> ()
              }
              frame #4 {
                n741 = local read "Sensor value"() -> (→"Air 0deg temp":dbl)
              }
            }
          }
          frame #1 {
            n742 = local write "Tab Control 4"(T12."Air Step 3" ("Tab Control 4")) -> ()
          }
        }
      }
      event "Temperature Continue Step 3": Value Change {
        n743 = event-data() -> ()  [unwired: 1 in, 6 out]
        n744 = stacked-sequence {
          frame #0 {
            n745 = stacked-sequence {
              frame #0 {
                n746 = Wait (ms)(milliseconds to wait=u32 1500) -> ()  [unwired: 1 out]
              }
              frame #1 {
              }
              frame #2 {
              }
              frame #3 {
                # "CAL;A1;<true_T>"
                n747 = local write "Due Write"("CAL;A1;60" ("Command")) -> ()
              }
              frame #4 {
                n748 = Wait (ms)(milliseconds to wait=u32 1000) -> ()  [unwired: 1 out]
              }
              frame #5 {
                # "CAL;A1;<true_T>"
                n749 = local read "Sensor value"() -> (→"Sample 60deg temp":dbl)
                n750 = local write "Due Write"("CAL;A1;60" ("Command")) -> ()
              }
            }
          }
          frame #1 {
            n751 = local read "Sample 0deg temp"() -> (w804:dbl)
            n752 = local read "Sample 60deg temp"() -> (w803:dbl)
            n753 = Add(x=w803, y="Temperature diff") -> (x+y=w801:dbl)
            n754 = Subtract(x=w803, y="Temperature diff") -> (x-y=w800:dbl)
            n755 = Add(x=w804, y="Temperature diff") -> (x+y=w799:dbl)
            n756 = Subtract(x=w804, y="Temperature diff") -> (x-y=w798:dbl)
            n757 = In Range and Coerce(upper limit=w801, x=w803, lower limit=w800) -> (In Range?=w797:bool)  [unwired: 1 out]
            n758 = In Range and Coerce(upper limit=w799, x=w804, lower limit=w798) -> (In Range?=w796:bool)  [unwired: 1 out]
            n759 = And(x=w797, y=w796) -> (x .and. y?=w795:bool)
            n760 = case shown="True" w795 {
              frame False {
                n761 = property on="Accept & Save sample Temperature step 4" class="Bool (strict)"("DisabledEnum"=T19."Disabled" ("Disabled")) -> ()  [unwired: 2 in, 2 out]
                n762 = local write "Sample Temperature Calibration"(enum32{"True", "Fail"}."Fail" ("Sample Temperature Calibration  2")) -> ()
              }
              frame True {
                n763 = property on="Accept & Save sample Temperature step 4" class="Bool (strict)"("DisabledEnum"=T19."Enabled" ("Disabled")) -> ()  [unwired: 2 in, 2 out]
                n764 = local write "Sample Temperature Calibration"(enum32{"True", "Fail"}."True" ("Sample Temperature Calibration  2")) -> ()
              }
            }
          }
          frame #2 {
          }
          frame #3 {
          }
          frame #4 {
          }
          frame #5 {
          }
          frame #6 {
            # "CAL;END"
          }
          frame #7 {
          }
          frame #8 {
            # "CAL;END"
          }
          frame #9 {
            n765 = local write "Tab Control 4"(T12."Step 4" ("Tab Control 4")) -> ()
          }
        }
      }
      event "Accept & Save sample Temperature step 4": Value Change {
        n766 = event-data() -> ()  [unwired: 1 in, 6 out]
        n767 = stacked-sequence {
          frame #0 {
            n768 = local write "Due Write"("CAL;SAVE" ("Command")) -> ()
          }
          frame #1 {
            n769 = Wait (ms)(milliseconds to wait=u32 1000) -> ()  [unwired: 1 out]
          }
          frame #2 {
            n770 = local write "Due Write"("CAL;SAVE" ("Command")) -> ()
          }
          frame #3 {
            n771 = Wait (ms)(milliseconds to wait=u32 1000) -> ()  [unwired: 1 out]
          }
          frame #4 {
            n772 = local write "Due Write"("CAL;END" ("Command")) -> ()
          }
          frame #5 {
            n773 = Wait (ms)(milliseconds to wait=u32 1000) -> ()  [unwired: 1 out]
          }
          frame #6 {
            n774 = local write "Due Write"("CAL;END" ("Command")) -> ()
            n775 = local write "Temperature Selection"(T13."Default" ("Temperature Selection")) -> ()
            n776 = local write "Calibration Selection"(T8."Default" ("Calibration Selection")) -> ()
            n777 = local write "Tab Control 4"(T12."Main" ("Tab Control 4")) -> ()
            n778 = local write "Main Calibration Tab"(T7."Temperature" ("Main Calibration Tab")) -> ()
          }
          frame #7 {
            n779 = Get Date/Time In Seconds() -> (seconds since 1Jan1904=w823:timestamp)
            n780 = Format Into String(format string="%<%I:%M:%S:%p %d:%B:%Y>T", w823) -> (resulting string=w821:string)  [unwired: 2 in, 1 out]
            n781 = local write "TEMPERATURE CALIBRATION"(w821) -> ()
          }
          frame #8 {
            n782 = local write "Save Button"(TRUE ("Save Button")) -> ()
          }
        }
      }
      event "Accept & Save Air Temperature step 4": Value Change {
        n783 = event-data() -> ()  [unwired: 1 in, 6 out]
        n784 = stacked-sequence {
          frame #0 {
            n785 = local write "Due Write"("CAL;SAVE" ("Command")) -> ()
          }
          frame #1 {
            n786 = Wait (ms)(milliseconds to wait=u32 1000) -> ()  [unwired: 1 out]
          }
          frame #2 {
            n787 = local write "Due Write"("CAL;SAVE" ("Command")) -> ()
          }
          frame #3 {
            n788 = Wait (ms)(milliseconds to wait=u32 1000) -> ()  [unwired: 1 out]
          }
          frame #4 {
            n789 = local write "Due Write"("CAL;END" ("Command")) -> ()
          }
          frame #5 {
            n790 = Wait (ms)(milliseconds to wait=u32 1000) -> ()  [unwired: 1 out]
          }
          frame #6 {
            n791 = local write "Due Write"("CAL;END" ("Command")) -> ()
            n792 = local write "Tab Control 4"(T12."Main" ("Tab Control 4")) -> ()
            n793 = local write "Main Calibration Tab"(T7."Temperature" ("Main Calibration Tab")) -> ()
            n794 = local write "Temperature Selection"(T13."Default" ("Temperature Selection")) -> ()
            n795 = local write "Calibration Selection"(T8."Default" ("Calibration Selection")) -> ()
          }
          frame #7 {
            n796 = Get Date/Time In Seconds() -> (seconds since 1Jan1904=w838:timestamp)
            n797 = Format Into String(format string="%<%I:%M:%S:%p %d:%B:%Y>T", w838) -> (resulting string=w837:string)  [unwired: 2 in, 1 out]
            n798 = local write "TEMPERATURE CALIBRATION"(w837) -> ()
          }
          frame #8 {
            n799 = local write "Save Button"(TRUE ("Save Button")) -> ()
          }
        }
      }
      event "Temperature Continue Step 6": Value Change {
        n800 = event-data() -> ()  [unwired: 1 in, 6 out]
        n801 = stacked-sequence {
          frame #0 {
            n802 = stacked-sequence {
              frame #0 {
                n803 = Wait (ms)(milliseconds to wait=u32 1000) -> ()  [unwired: 1 out]
              }
              frame #1 {
              }
              frame #2 {
              }
              frame #3 {
                # "CAL;A1;<true_T>"
                n804 = local write "Due Write"("CAL;A1;60" ("Command")) -> ()
              }
              frame #4 {
                n805 = Wait (ms)(milliseconds to wait=u32 1000) -> ()  [unwired: 1 out]
              }
              frame #5 {
                # "CAL;A1;<true_T>"
                n806 = local write "Due Write"("CAL;A1;60" ("Command")) -> ()
              }
            }
          }
          frame #1 {
            n807 = local read "Sensor value"() -> (→"Air 60deg temp":dbl)
          }
          frame #2 {
          }
          frame #3 {
          }
          frame #4 {
          }
          frame #5 {
          }
          frame #6 {
            # "CAL;END"
          }
          frame #7 {
            n808 = local read "Temperature diff"() -> (w847:dbl)
            n809 = local read "Air 60deg temp"() -> (w846:dbl)
            n810 = local read "Air 0deg temp"() -> (w845:dbl)
            n811 = Add(x=w846, y=w847) -> (x+y=w854:dbl)
            n812 = Subtract(x=w846, y=w847) -> (x-y=w853:dbl)
            n813 = Add(x=w845, y=w847) -> (x+y=w852:dbl)
            n814 = Subtract(x=w845, y=w847) -> (x-y=w851:dbl)
            n815 = In Range and Coerce(upper limit=w854, x=w846, lower limit=w853) -> (In Range?=w850:bool)  [unwired: 1 out]
            n816 = In Range and Coerce(upper limit=w852, x=w845, lower limit=w851) -> (In Range?=w849:bool)  [unwired: 1 out]
            n817 = And(x=w850, y=w849) -> (x .and. y?=w848:bool)
            n818 = case shown="True" w848 {
              frame False {
                n819 = property on="Accept & Save Air Temperature step 4" class="Bool (strict)"("DisabledEnum"=T19."Disabled" ("Disabled")) -> ()  [unwired: 2 in, 2 out]